vi "labHolo.vi"() -> ()   [LabVIEW 2023] (continued)
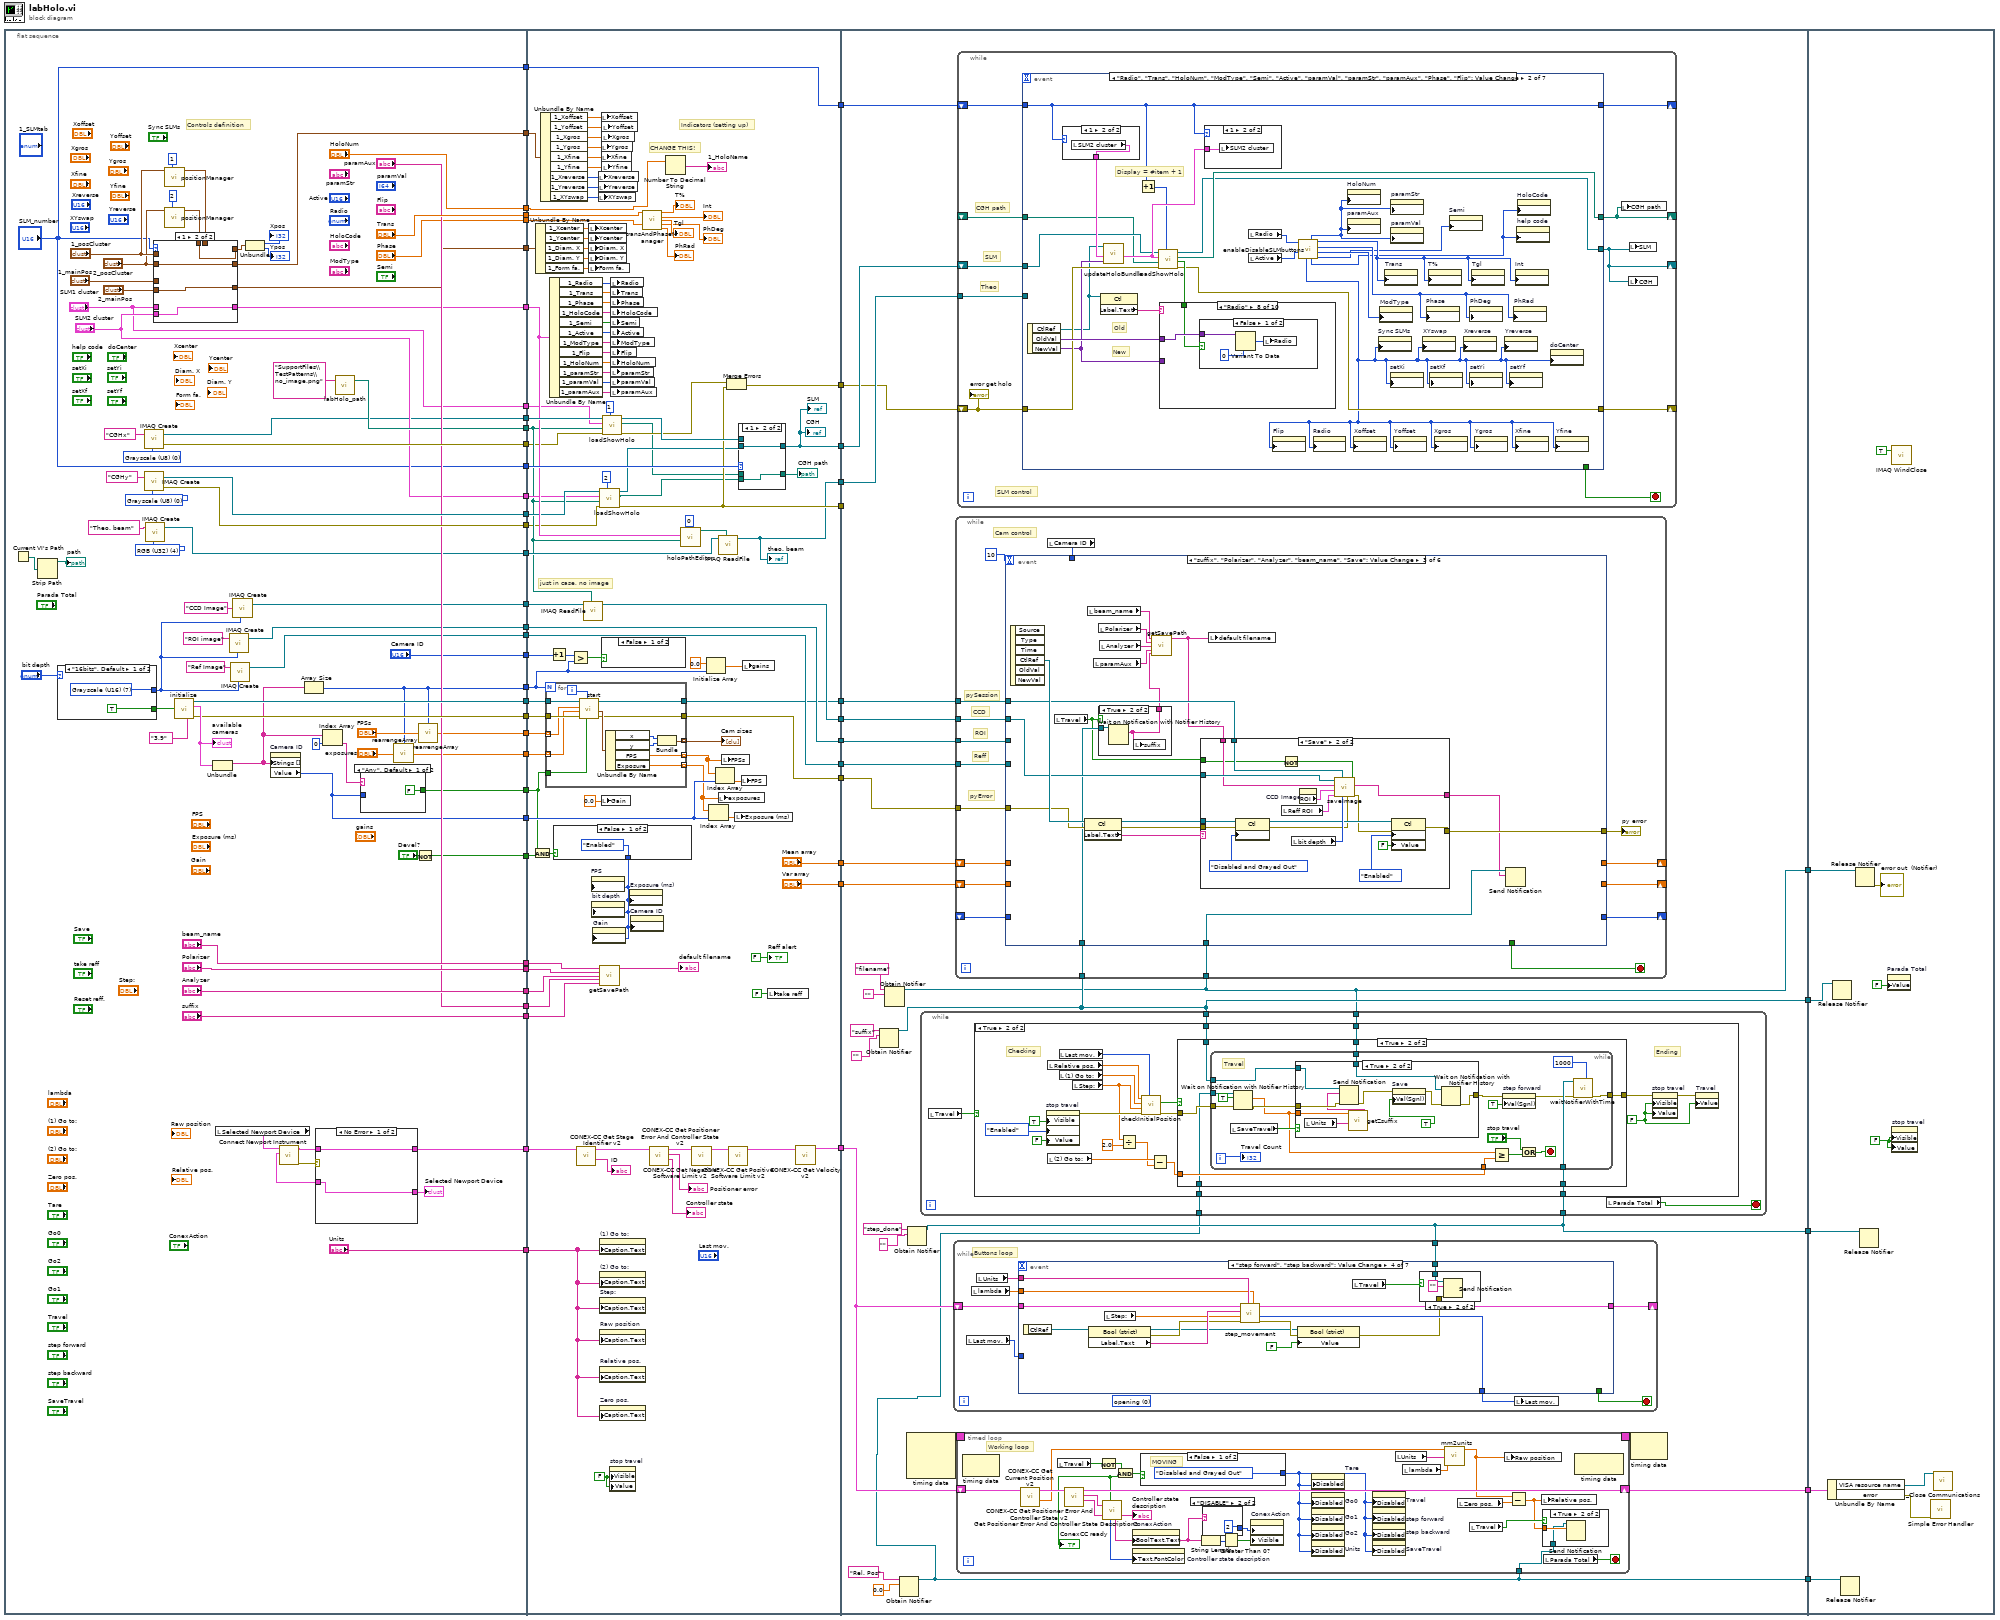
[diagram p0: block diagram]
diagram:
  n1 = flat-sequence {
    tunnel: [w77] -> w53
    tunnel: [w124] -> w52
    tunnel: [w123] -> w51
    tunnel: [w122] -> w50
    tunnel: ["Trans"] -> w47
    tunnel: ["Phase"] -> w46
    tunnel: [w114] -> w45
    tunnel: [w71] -> w44
    tunnel: [w113] -> w43
    tunnel: ["beam_name"] -> w42
    tunnel: ["Polarizer"] -> w41
    tunnel: ["Analyzer"] -> w40
    tunnel: ["suffix"] -> w39
    tunnel: ["paramAux"] -> w38
    tunnel: [w105] -> w37
    tunnel: [w104] -> w35
    tunnel: [w101] -> w33
    tunnel: [w97] -> w32
    tunnel: [w96] -> w31
    tunnel: [w83] -> w30
    tunnel: ["HoloNum"] -> w29
    tunnel: ["SLM1 cluster"] -> w28
    tunnel: [w81] -> w27
    tunnel: ["SLM2 cluster"] -> w26
    tunnel: ["SLM_number"] -> w25
    tunnel: [w74] -> w24
    tunnel: [w65] -> w18
    tunnel: [w63] -> w16
    tunnel: [w70] -> w15
    tunnel: [w68] -> w14
    tunnel: [w66] -> w13
    tunnel: ["Camera ID"] -> w12
    tunnel: ["SLM_number"] -> w10
    tunnel: ["Units"] -> w8
    tunnel: [w57] -> w5
    tunnel: w53 -> [w255]
    tunnel: w52 -> [w200]
    tunnel: w51 -> [w197]
    tunnel: w50 -> [w196]
    tunnel: [w244] -> w49
    tunnel: [w183] -> w48
    tunnel: w47 -> [w249]
    tunnel: w46 -> [w248]
    tunnel: w45 -> [w184]
    tunnel: w44 -> [w181]
    tunnel: w43 -> [w185]
    tunnel: w42 -> [w189]
    tunnel: w41 -> [w188]
    tunnel: w40 -> [w187]
    tunnel: w39 -> [w246]
    tunnel: w38 -> [w186]
    tunnel: w37 -> [w245]
    tunnel: [w243] -> w36
    tunnel: w35 -> [w243]
    tunnel: [w240] -> w34
    tunnel: w33 -> [w240]
    tunnel: w32 -> [w224]
    tunnel: w31 -> [w230]
    tunnel: w30 -> [w207]
    tunnel: w29 -> [w210]
    tunnel: w28 -> [w203]
    tunnel: w27 -> [w198]
    tunnel: w26 -> [w199]
    tunnel: w25 -> [w209]
    tunnel: w24 -> [w208]
    tunnel: [w192] -> w23
    tunnel: [w195] -> w22
    tunnel: [w162] -> w21
    tunnel: ["Mean array"] -> w20
    tunnel: ["Var array"] -> w19
    tunnel: w18 -> [w166]
    tunnel: [w176] -> w17
    tunnel: w16 -> [w175]
    tunnel: w15 -> [w170]
    tunnel: w14 -> [w169]
    tunnel: w13 -> [w174]
    tunnel: w12 -> [w164]
    tunnel: [w158] -> w11
    tunnel: w10 -> [w157]
    tunnel: [w157] -> w9
    tunnel: w8 -> [w155]
    tunnel: [w154] -> w7
    tunnel: w5 -> [w153]
    tunnel: w49 -> [w303]
    tunnel: w48 -> [w302]
    tunnel: w36 -> [w301]
    tunnel: w34 -> [w300]
    tunnel: w23 -> [w296]
    tunnel: w22 -> [_]
    tunnel: w21 -> [w295]
    tunnel: w20 -> [w299]
    tunnel: w19 -> [w298]
    tunnel: w17 -> [w297]
    tunnel: w11 -> [w294]
    tunnel: w9 -> [w293]
    tunnel: w7 -> [w289]
    tunnel: [w290] -> w6
    tunnel: [w282] -> w4
    tunnel: [w281] -> w3
    tunnel: [w280] -> w2
    tunnel: [w277] -> w1
    tunnel: w6 -> [w958]
    tunnel: w4 -> [w955]
    tunnel: w3 -> [w954]
    tunnel: w2 -> [w953]
    tunnel: w1 -> [w952]
    frame #0 {
      w75 = T15 4 items=["Grayscale (U8)", "Grayscale (I16)", "Grayscale (SGL)", "Complex (CSG)", "RGB (U32)", "HSL (U32)", "RGB (U64)", "Grayscale (U16)"] ("Image Type")
      w117 = T15 0 items=["Grayscale (U8)", "Grayscale (I16)", "Grayscale (SGL)", "Complex (CSG)", "RGB (U32)", "HSL (U32)", "RGB (U64)", "Grayscale (U16)"] ("Image Type")
      w118 = T15 0 items=["Grayscale (U8)", "Grayscale (I16)", "Grayscale (SGL)", "Complex (CSG)", "RGB (U32)", "HSL (U32)", "RGB (U64)", "Grayscale (U16)"] ("Image Type")
      # "Controls definition"
      n2 = Current VI's Path() -> (path=w121:path)
      n3 = Strip Path(path=w121) -> (stripped path=→"path":path)  [unwired: 1 out]
      n4 = case shown="\"16bits\", Default" "bit depth" {
        tunnel: [w143 w145] -> w102
        tunnel: [TRUE FALSE] -> w107
        frame "16bits", Default {
          w143 = T15 7 items=["Grayscale (U8)", "Grayscale (I16)", "Grayscale (SGL)", "Complex (CSG)", "RGB (U32)", "HSL (U32)", "RGB (U64)", "Grayscale (U16)"] ("Image Type")
        }
        frame "8bits" {
          w145 = T15 0 items=["Grayscale (U8)", "Grayscale (I16)", "Grayscale (SGL)", "Complex (CSG)", "RGB (U32)", "HSL (U32)", "RGB (U64)", "Grayscale (U16)"] ("Image Type")
        }
      }
      n5 = call "IMAQ Create"("Image Name"="CGHx", "Image Type"=w118) -> ("New Image"=w77:T6, "error out"=w122:errorcluster)  [unwired: 3 in]
      n6 = call "IMAQ Create"("Image Name"="CGHy", "Image Type"=w117) -> ("New Image"=w124:T6, "error out"=w123:errorcluster)  [unwired: 3 in]
      n7 = call "IMAQ Create"("Image Name"="Theo. beam", "Image Type"=w75) -> ("New Image"=w74:T6)  [unwired: 3 in, 1 out]
      n8 = call "positionManager.vi"("Display"=1, "Cluster"="1_posCluster") -> ("output cluster"=w89:cluster{i32, i32})  [unwired: 5 in, 2 out]
      n9 = call "positionManager.vi"("Display"=2, "Cluster"="2_posCluster") -> ("output cluster"=w90:cluster{i32, i32})  [unwired: 5 in, 2 out]
      n10 = case shown="1" "SLM_number" {
        tunnel: [w135 w137] -> w97
        tunnel: [w134 w139] -> w96
        tunnel: "1_posCluster" -> [w135 _]
        tunnel: "1_mainPos" -> [w134 _]
        tunnel: "2_posCluster" -> [_ w137]
        tunnel: "2_mainPos" -> [_ w139]
        tunnel: "SLM1 cluster" -> [w133 _]
        tunnel: "SLM2 cluster" -> [_ w138]
        tunnel: [w133 w138] -> w83
        tunnel: [w132 w136] -> w84
        tunnel: w90 -> [_ w136]
        tunnel: w89 -> [w132 _]
        frame 0, Default {
        }
        frame 1 {
        }
      }
      n11 = call "initialize.vi"("14bits"=w107, "sys Python version"="3.9") -> ("session out"=w113:refnum<k35>, "available cameras"=w115:cluster{string[], string[]}, "error out"=w114:errorcluster)  [unwired: 2 in]
      "available\ncameras" <- w115
      n12 = Unbundle(w115) -> (w99:string[])  [unwired: 1 out]
      n13 = local read "Selected Newport Device"() -> (w59:T1)
      n14 = call "IMAQ Create"("Image Name"="ROI image", "Image Type"=w102) -> ("New Image"=w101:T6)  [unwired: 3 in, 1 out]
      n15 = call "IMAQ Create"("Image Name"="Ref Image", "Image Type"=w102) -> ("New Image"=w104:T6)  [unwired: 3 in, 1 out]
      n16 = call "IMAQ Create"("Image Name"="CCD Image", "Image Type"=w102) -> ("New Image"=w105:T6)  [unwired: 3 in, 1 out]
      n17 = Unbundle(w84) -> (→"Xpos":i32, →"Ypos":i32)
      n18 = property on="Camera ID" class="Ring (strict)"("Strings []"=w99) -> ("Value"=w71:u16)  [unwired: 2 in, 2 out]
      n19 = call "Connect Newport Instrument.vi"("Selected Device Cluster (INPUT)"=w59) -> ("error (duplicate)"=w58:errorcluster, "Device Connection Cluster"=w56:T16, "Selected Device Cluster (OUTPUT)"=w55:T1)  [unwired: 5 in, 3 out]
      n20 = Array Size(array=w99) -> (size(s)=w65:i32)
      n21 = case shown="No Error" w58 {
        tunnel: [w128 w131] -> w57
        tunnel: w56 -> [w128 _]
        tunnel: w55 -> [w127 _]
        tunnel: [w127 w129] -> w54
        frame No Error {
        }
        frame Error {
          n22 = call "Connect Newport Instrument.vi"("Selected Device Cluster (INPUT)"=T10 {"Found resources names"=["ASRL1::INSTR", "ASRL3::INSTR"], "Found interfaces names"=["ASRL1  (COM1 - Puerto de comunicaciones)", "ASRL3  (COM3 - USB Serial Port)"], "OK?"=FALSE, "Selected device"="", "Address"=0, "error"={"status"=TRUE, "code"=0, "source"=""}}) -> ("Device Connection Cluster"=w131:T16, "Selected Device Cluster (OUTPUT)"=w129:T1)  [unwired: 5 in, 4 out]
        }
      }
      "Selected Newport Device" <- w54
      n23 = Index Array(array=w99, index=0) -> (element=w100:string)
      n24 = call "labHolo_path.vi"("sub folder or file (str)"="SupportFiles\\TestPatterns\\no_image.png") -> ("labHolo path"=w81:path)  [unwired: 1 in, 1 out]
      n25 = case shown="\"Any\", Default" w100 {
        tunnel: w71 -> [_ _]
        tunnel: [FALSE TRUE] -> w70
        frame "Any", Default {
        }
        frame "NotFound" {
        }
      }
      n26 = call "rearrengeArray.vi"("array in"="exposures", "desired size"=w65) -> ("array out"=w63:dbl[])
      n27 = Not(x="Devel?") -> (.not. x?=w68:bool)
      n28 = call "rearrengeArray.vi"("array in"="FPSs", "desired size"=w65) -> ("array out"=w66:dbl[])
    }
    frame #1 {
      w146 = FALSE ("Visible")
      # "just in case, no image"
      # "CHANGE THIS!"
      # "Indicators (setting up)"
      n29 = And(x=w170, y=w169) -> (x .and. y?=w171:bool)
      n30 = Unbundle By Name(w230) -> ("1_Xcenter"=w229:dbl, "1_Ycenter"=w228:dbl, "1_Diam. X"=w227:dbl, "1_Diam. Y"=w226:dbl, "1_Form fa."=w225:dbl)
      n31 = Unbundle By Name(w224) -> ("1_Xoffset"=w239:dbl, "1_Yoffset"=w238:dbl, "1_Xgros"=w237:dbl, "1_Ygros"=w236:dbl, "1_Xfine"=w235:dbl, "1_Yfine"=w234:dbl, "1_Xreverse"=w233:u16, "1_Yreverse"=w232:u16, "1_XYswap"=w231:u16)
      n32 = for {
        N: w166 -> [_]
        tunnel: w185 -> [w272]
        tunnel: w184 -> [w271]
        tunnel: [w270] -> w183
        tunnel: [w269] -> w179 mode=indexing
        tunnel: [w268] -> w180 mode=indexing
        tunnel: [w266] -> w177 mode=indexing
        tunnel: [w265] -> w176
        tunnel: w174 -> [w264] mode=indexing
        tunnel: w175 -> [w263] mode=indexing
        tunnel: w170 -> [w259]
        i -> [w262]
        n33 = call "start.vi"("Not found"=w259, "Cam id"=w262, "error in (no error)"=w271, "Exposure (ms)"=w263, "FPS"=w264, "session in"=w272) -> ("error out"=w265:errorcluster, "cam attr."=w267:T17, "session out"=w270:refnum<k35>)  [unwired: 2 in]
        n34 = Unbundle By Name(w267) -> ("x"=w261:i32, "y"=w260:i32, "FPS"=w269:dbl, "Exposure"=w268:dbl)
        n35 = Bundle("x"=w261, "y"=w260) -> (w266:cluster{"x":i32, "y":i32})  [unwired: 1 in]
      }
      "Cam sizes" <- w177
      n36 = Unbundle By Name(w207) -> ("1_Radio"=w223:T7, "1_Trans"=w222:dbl, "1_Phase"=w221:dbl, "1_HoloCode"=w220:string, "1_Semi"=w219:bool, "1_Active"=w218:u16, "1_ModType"=w217:string, "1_Flip"=w216:string, "1_HoloNum"=w215:dbl, "1_paramStr"=w214:string, "1_paramVal"=w213:i64, "1_paramAux"=w212:string)
      n37 = Increment(x=w164) -> (x+1=w165:u16)
      n38 = case shown="False" w171 {
        tunnel: [T11."Enabled" ("Disabled") T11."Disabled and Grayed Out" ("Disabled")] -> w163
        frame False {
        }
        frame True {
        }
      }
      n39 = Greater?(x=w165, y=w166) -> (0:w167:bool)
      n40 = call "CONEX-CC Get Stage Identifier v2.vi"("Connection Cluster in"=w153) -> ("Identifier"=→"ID":string, "Connection Cluster out"=w149:T16)  [unwired: 9 in]
      n41 = call "IMAQ ReadFile"("File Path"=w198, "Image"=w245) -> ("Image Out"=w244:T6)  [unwired: 5 in, 4 out]
      n42 = local write "Xcenter"(w229) -> ()
      n43 = local write "Ycenter"(w228) -> ()
      n44 = local write "Diam. X"(w227) -> ()
      n45 = local write "Diam. Y"(w226) -> ()
      n46 = local write "Form fa."(w225) -> ()
      n47 = property on="FPS" class="DigNum (strict)"("DisabledEnum"=w163) -> ()  [unwired: 2 in, 2 out]
      n48 = property on="bit depth" class="Enum (strict)"("DisabledEnum"=w163) -> ()  [unwired: 2 in, 2 out]
      n49 = property on="Gain" class="DigNum (strict)"("DisabledEnum"=w163) -> ()  [unwired: 2 in, 2 out]
      n50 = local write "Xreverse"(w233) -> ()
      n51 = local write "Yreverse"(w232) -> ()
      n52 = local write "XYswap"(w231) -> ()
      n53 = call "loadShowHolo.vi"("Display"=u16 2, "error in (no error)"=w197, "prev. path"=w198, "SLM1 cluster"=w199, "Image in"=w200) -> ("error out"=w195:errorcluster, "appended path"=w159:path, "Image out"=w193:T6)  [unwired: 3 in, 1 out]
      n54 = call "getSavePath.vi"("beam_name"=w189, "Polarizer"=w188, "Analyzer"=w187, "prefix"=w186, "suffix"=w246) -> ("appended filename"=→"default filename":string)  [unwired: 10 in]
      n55 = property on="(1) Go to:" class="DigNum (strict)"("Caption.Text"=w155) -> ()  [unwired: 2 in, 2 out]
      n56 = property on="(2) Go to:" class="DigNum (strict)"("Caption.Text"=w155) -> ()  [unwired: 2 in, 2 out]
      n57 = property on="Step:" class="DigNum (strict)"("Caption.Text"=w155) -> ()  [unwired: 2 in, 2 out]
      n58 = property on="Raw position" class="DigNum (strict)"("Caption.Text"=w155) -> ()  [unwired: 2 in, 2 out]
      n59 = property on="Relative pos." class="DigNum (strict)"("Caption.Text"=w155) -> ()  [unwired: 2 in, 2 out]
      n60 = property on="Zero pos." class="DigNum (strict)"("Caption.Text"=w155) -> ()  [unwired: 2 in, 2 out]
      n61 = local write "Xoffset"(w239) -> ()
      n62 = local write "Ygros"(w236) -> ()
      n63 = local write "Xfine"(w235) -> ()
      n64 = local write "Gain"(0.0 ("Gain")) -> ()
      n65 = local write "Yoffset"(w238) -> ()
      n66 = local write "Xgros"(w237) -> ()
      n67 = local write "Yfine"(w234) -> ()
      n68 = case shown="False" w167 {
        frame False {
        }
        frame True {
          n69 = local write "Camera ID"(u16 0) -> ()
        }
      }
      n70 = call "loadShowHolo.vi"("Display"=u16 1, "error in (no error)"=w196, "prev. path"=w198, "SLM1 cluster"=w203, "Image in"=w255) -> ("error out"=w161:errorcluster, "appended path"=w160:path, "Image out"=w202:T6)  [unwired: 3 in, 1 out]
      n71 = property on="stop travel" class="Bool (strict)"("Visible"=w146, "Value"=w146) -> ()  [unwired: 2 in, 2 out]
      n72 = local write "Radio"(w223) -> ()
      n73 = local write "Trans"(w222) -> ()
      n74 = local write "Phase"(w221) -> ()
      n75 = local write "HoloCode"(w220) -> ()
      n76 = local write "Semi"(w219) -> ()
      n77 = local write "Active"(w218) -> ()
      n78 = local write "ModType"(w217) -> ()
      n79 = local write "Flip"(w216) -> ()
      n80 = local write "HoloNum"(w215) -> ()
      n81 = local write "paramStr"(w214) -> ()
      n82 = local write "paramVal"(w213) -> ()
      n83 = local write "paramAux"(w212) -> ()
      n84 = property on="Exposure (ms)" class="DigNum (strict)"("DisabledEnum"=w163) -> ()  [unwired: 2 in, 2 out]
      n85 = property on="Camera ID" class="Ring (strict)"("DisabledEnum"=w163) -> ()  [unwired: 2 in, 2 out]
      n86 = call "transAndPhaseManager.vi"("Trans in"=w249, "Phase in"=w248) -> ("Trans %"=→"T%":dbl, "Intensity"=→"Int":dbl, "T gl"=→"Tgl":dbl, "Phase Deg"=→"PhDeg":dbl, "Phase Rad"=→"PhRad":dbl)  [unwired: 9 in]
      n87 = call "CONEX-CC Get Positioner Error And Controller State v2.vi"("Connection Cluster in"=w149) -> ("Controller state"=→"Controller state":string, "Positioner error"=→"Positioner error":string, "Connection Cluster out"=w148:T16)  [unwired: 8 in]
      n88 = Number To Decimal String(number=w210) -> (decimal integer string=→"1_HoloName":string)  [unwired: 1 in]
      n89 = call "holoPathEditor.vi"("Display"=u16 0, "prev. Path"=w198, "input cluster"=w207) -> ("appended path"=w206:path)  [unwired: 5 in, 3 out]
      n90 = call "CONEX-CC Get Negative Software Limit v2.vi"("Connection Cluster in"=w148) -> ("Connection Cluster out"=w147:T16)  [unwired: 9 in, 1 out]
      n91 = Initialize Array(0.0 ("element"), w166) -> (w173:dbl[])
      n92 = Index Array(array=w180, index=w181) -> (element=w178:dbl)
      n93 = Index Array(array=w179, index=w181) -> (element=w182:dbl)
      n94 = call "IMAQ ReadFile"("File Path"=w206, "Image"=w208) -> ("Image Out"=w162:T6)  [unwired: 5 in, 4 out]
      "theo. beam" <- w162
      n95 = local write "exposures"(w180) -> ()
      n96 = local write "FPSs"(w179) -> ()
      n97 = Merge Errors(w161, w195) -> (w158:errorcluster)
      n98 = call "CONEX-CC Get Positive Software Limit v2.vi"("Connection Cluster in"=w147) -> ("Connection Cluster out"=w156:T16)  [unwired: 9 in, 1 out]
      n99 = local write "Exposure (ms)"(w178) -> ()
      n100 = case shown="1" w209 {
        tunnel: [w274 w276] -> w192
        tunnel: w202 -> [w274 _]
        tunnel: w160 -> [w273 _]
        tunnel: [w273 w275] -> w194
        tunnel: w193 -> [_ w276]
        tunnel: w159 -> [_ w275]
        frame 0, Default {
        }
        frame 1 {
        }
      }
      "CGH path" <- w194
      "CGH" <- w192
      "SLM" <- w192
      n101 = local write "FPS"(w182) -> ()
      n102 = local write "gains"(w173) -> ()
      n103 = local write "take reff"(FALSE ("take reff")) -> ()
      n104 = call "CONEX-CC Get Velocity v2.vi"("Connection Cluster in"=w156) -> ("Connection Cluster out"=w154:T16)  [unwired: 8 in, 2 out]
      "Reff alert" <- FALSE ("Boolean")
    }
    frame #2 {
      n105 = Obtain Notifier(name (unnamed)="suffix", notification data type="") -> (notifier out=w281:refnum<notifier>)  [unwired: 2 in, 2 out]
      n106 = Obtain Notifier(name (unnamed)="filename", notification data type="") -> (notifier out=w280:refnum<notifier>)  [unwired: 2 in, 2 out]
      n107 = Obtain Notifier(name (unnamed)="Rel. Pos", notification data type=0.0) -> (notifier out=w277:refnum<notifier>)  [unwired: 2 in, 2 out]
      n108 = node-c288() -> (w292:T12)  [unwired: 2 in, 1 out]
      n109 = Obtain Notifier(name (unnamed)="step_done", notification data type="") -> (notifier out=w282:refnum<notifier>)  [unwired: 2 in, 2 out]
      n110 = while {
        tunnel: w281 -> [w307]
        tunnel: w282 -> [w306]
        tunnel: w280 -> [w305]
        tunnel: w277 -> [w304]
        stop <- w308 stop-if-true
        n111 = local read "Travel"() -> (w309:bool)
        n112 = case shown="True" w309 {
          tunnel: w307 -> [_ w330]
          tunnel: w306 -> [_ w329]
          tunnel: w305 -> [_ w311]
          tunnel: w304 -> [_ w310]
          frame False {
          }
          frame True {
            w318 = FALSE ("Visible")
            # "Ending"
            # "Checking"
            n113 = property on="stop travel" class="Bool (strict)"("Visible"=TRUE, "DisabledEnum"=T11."Enabled" ("Disabled"), "Value"=FALSE ("stop travel")) -> (error out=w325:errorcluster)  [unwired: 2 in, 1 out]
            n114 = local read "Relative pos."() -> (w322:dbl)
            n115 = local read "(2) Go to:"() -> (w316:dbl)
            n116 = local read "Last mov."() -> (w323:u16)
            n117 = local read "(1) Go to:"() -> (w324:dbl)
            n118 = local read "Step:"() -> (w314:dbl)
            n119 = Divide(x=w314, y=2.0) -> (x/y=w312:dbl)
            n120 = call "checkInitialPosition.vi"("Last mov."=w323, "error in (no error)"=w325, "Step"=w314, "Initial pos"=w324, "Current pos"=w322) -> ("error out"=w321:errorcluster, "go"=w317:bool)  [unwired: 5 in]
            n121 = Subtract(x=w316, y=w312) -> (x-y=w315:dbl)
            n122 = case shown="True" w317 {
              tunnel: w330 -> [_ w338]
              tunnel: w329 -> [_ w337]
              tunnel: w321 -> [w331 w336]
              tunnel: [w331 w335] -> w320
              tunnel: w315 -> [_ w334]
              tunnel: w311 -> [_ w333]
              tunnel: w310 -> [_ w332]
              frame False {
              }
              frame True {
                n123 = while {
                  tunnel: w338 -> [w354]
                  tunnel: w337 -> [w343]
                  tunnel: w336 -> [w347]
                  tunnel: [w341] -> w335
                  tunnel: w334 -> [w352]
                  tunnel: w333 -> [w348]
                  tunnel: w332 -> [w345]
                  i -> [w353]
                  stop <- w357 stop-if-true
                  # "Travel"
                  n124 = local read "SaveTravel"() -> (w356:bool)
                  n125 = Wait on Notification with Notifier History(0:w345, 1:TRUE ("ignore previous (F)"), 3:w347) -> (9:w344:dbl, 11:w346:errorcluster)  [unwired: 1 in, 2 out]
                  n126 = case shown="True" w356 {
                    tunnel: w346 -> [w358 w364]
                    tunnel: [w358 w359] -> w349
                    tunnel: w354 -> [_ w362]
                    tunnel: w344 -> [_ w366]
                    tunnel: w348 -> [_ w361]
                    frame False {
                    }
                    frame True {
                      n127 = local read "Units"() -> (w367:string)
                      n128 = call "getZsuffix.vi"("Units"=w367, "Zposition"=w366) -> ("String"=w363:string)  [unwired: 9 in]
                      n129 = Send Notification(notification=w363, notifier=w362, error in (no error)=w364) -> (error out=w365:errorcluster)  [unwired: 1 out]
                      n130 = property on="Save" class="Bool (strict)"(error in=w365, "Val(Sgnl)"=TRUE ("Value (Signaling)")) -> (error out=w360:errorcluster)  [unwired: 1 in, 1 out]
                      n131 = Wait on Notification with Notifier History(0:w361, 3:w360) -> (11:w359:errorcluster)  [unwired: 2 in, 3 out]
                    }
                  }
                  n132 = Greater Or Equal?(x=w344, y=w352) -> (x >= y?=w350:bool)
                  n133 = property on="step forward" class="Bool (strict)"(error in=w349, "Val(Sgnl)"=TRUE ("Value (Signaling)")) -> (error out=w342:errorcluster)  [unwired: 1 in, 1 out]
                  n134 = Or(x="stop travel", y=w350) -> (x .or. y?=w357:bool)
                  n135 = call "waitNotifierWithTime.vi"("min wait in ms (500)"=u32 1000 ("min wait in ms (300)"), "error in (no error)"=w342, "Notifier in"=w343) -> ("error out"=w341:errorcluster)  [unwired: 6 in, 2 out]
                  "Travel Count" <- w353
                }
              }
            }
            n136 = property on="stop travel" class="Bool (strict)"(error in=w320, "Visible"=w318, "Value"=w318) -> (error out=w319:errorcluster)  [unwired: 1 in, 1 out]
            n137 = property on="Travel" class="Bool (strict)"(error in=w319, "Value"=w318) -> ()  [unwired: 1 in, 2 out]
          }
        }
        n138 = local read "Parada Total"() -> (w308:bool)
      }
      n139 = while {
        shift-right: [w409] -> _
        shift-left: w289 -> [w410]
        tunnel: w282 -> [w404]
        stop <- w411 stop-if-true
        (unwired) u16 0 items=["opening", "homing", "toLeft", "toRight", "closing"] ("Last movement")
        # "Buttons loop"
        n140 = local read "Last mov."() -> (w405:u16)
        n141 = local read "lambda"() -> (w407:dbl)
        n142 = local read "Units"() -> (w408:string)
        n143 = event shown="[3] \"step forward\", \"step backward\": Value Change" {
          selector: _ -> [_ _ _ _ _ _ _]
          dyn-events: _ -> [_ _ _ _ _ _ _]
          timeout: _ -> [_ _ _ _ _ _ _]
          tunnel: [_ w415 _ _ _ _ _] -> w411
          tunnel: w410 -> [_ w416 w434 w468 w488 w495 w506]
          tunnel: [_ w414 w433 w467 w487 w495 w506] -> w409
          tunnel: w408 -> [_ _ _ w461 w486 _ _]
          tunnel: w407 -> [_ _ _ w460 w485 _ w499]
          tunnel: [w412 w413 w429 w458 w477 w494 w498] -> w406
          tunnel: w405 -> [w412 w413 w428 _ _ w494 w498]
          tunnel: w404 -> [_ _ _ w459 _ _ _]
          event Timeout {
            n144 = event-data() -> ()  [unwired: 1 in, 3 out]
          }
          event "Parada Total": Value Change {
            n145 = event-data() -> ()  [unwired: 1 in, 1 out]
            n146 = flat-sequence {
              tunnel: [w421] -> w419
              tunnel: w416 -> [w420]
              tunnel: w419 -> [w423]
              tunnel: [w423] -> w418
              tunnel: w418 -> [w425]
              tunnel: [w425] -> w417
              tunnel: [w427] -> w414
              tunnel: w417 -> [w427]
              tunnel: [TRUE] -> w415
              frame #0 {
                n147 = call "CONEX-CC Stop Motion v2.vi"("Connection Cluster in"=w420) -> ("Connection Cluster out"=w421:T16)  [unwired: 10 in]
              }
              frame #1 {
                n148 = local write "Travel"(FALSE) -> ()
              }
              frame #2 {
                n149 = Wait (ms)(milliseconds to wait=u32 200 ("attente (ms)")) -> ()  [unwired: 1 out]
              }
              frame #3 {
              }
            }
          }
          event "ConexAction": Value Change {
            n150 = event-data() -> ("CtlRef"=w431:refnum<vi>)  [unwired: 1 in]
            n151 = property on="Property Node" class="Bool (strict)"(reference=w431) -> ("BoolText.Text"=w430:string)  [unwired: 1 in, 2 out]
            n152 = case shown="\"STOP\"" w430 {
              tunnel: w434 -> [w437 w440 w443 w451 w454]
              tunnel: [w436 w440 w442 w450 w455] -> w433
              tunnel: [w435 w439 w441 w448 w453] -> w429
              tunnel: w428 -> [w435 w439 _ w448 w453]
              frame "ENABLE" {
                n153 = call "CONEX-CC Enter-Leave DISABLE State v2.vi"("Ready? (false=DISABLE true=READY)"=TRUE ("Flag (false=DISABLE true=READY)"), "Connection Cluster in"=w437) -> ("Connection Cluster out"=w436:T16)  [unwired: 7 in]
              }
              frame Default {
              }
              frame "HOME" {
                n154 = flat-sequence {
                  tunnel: w443 -> [w447]
                  tunnel: [w446] -> w442
                  tunnel: [w445] -> w441
                  frame #0 {
                    n155 = One Button Dialog(message="The Stage will go to the 0 position. Check that the travel is clean!") -> ()  [unwired: 1 in, 1 out]
                  }
                  frame #1 {
                    w445 = u16 0 items=["opening", "homing", "toLeft", "toRight", "closing"] ("Last movement")
                    n156 = call "CONEX-CC Home search v2.vi"("Connection Cluster in"=w447) -> ("Connection Cluster out"=w446:T16)  [unwired: 5 in, 3 out]
                  }
                }
              }
              frame "DISABLE" {
                n157 = call "CONEX-CC Enter-Leave DISABLE State v2.vi"("Ready? (false=DISABLE true=READY)"=FALSE ("Flag (false=DISABLE true=READY)"), "Connection Cluster in"=w451) -> ("Connection Cluster out"=w450:T16)  [unwired: 7 in]
              }
              frame "STOP" {
                n158 = call "CONEX-CC Stop Motion v2.vi"("Connection Cluster in"=w454) -> ("Connection Cluster out"=w455:T16)  [unwired: 10 in]
                n159 = local write "stop travel"(TRUE ("stop travel")) -> ()
              }
            }
            n160 = property on="ConexAction" class="Bool (strict)"("Value"=FALSE) -> ()  [unwired: 2 in, 2 out]
          }
          event "step forward", "step backward": Value Change {
            n161 = event-data() -> ("CtlRef"=w470:refnum<vi>)  [unwired: 1 in]
            n162 = property on="Property Node" class="Bool (strict)"(reference=w470) -> (reference out=w463:refnum<vi>, error out=w465:errorcluster, "Label.Text"=w466:string)  [unwired: 1 in]
            n163 = local read "Step:"() -> (w462:dbl)
            n164 = call "step_movement.vi"("lambda (nm)"=w460, "Units"=w461, "error in (no error)"=w465, "step (units)"=w462, "Step type (fordward)"=w466, "Connection Cluster in"=w468) -> ("error out"=w464:errorcluster, "Last mov."=w458:u16, "Connection Cluster out"=w467:T16)  [unwired: 3 in]
            n165 = property on="Property Node" class="Bool (strict)"(reference=w463, error in=w464, "Value"=FALSE) -> (error out=w457:errorcluster)  [unwired: 1 out]
            n166 = local read "Travel"() -> (w456:bool)
            n167 = case shown="True" w456 {
              tunnel: w459 -> [_ w473]
              tunnel: w457 -> [_ w472]
              frame False {
              }
              frame True {
                n168 = Send Notification(notification="", notifier=w473, error in (no error)=w472) -> ()  [unwired: 2 out]
              }
            }
          }
          event "Go1", "Go2", "Go0": Value Change {
            n169 = event-data() -> ("CtlRef"=w484:refnum<vi>)  [unwired: 1 in]
            n170 = property on="Property Node" class="Bool (strict)"(reference=w484) -> (reference out=w483:refnum<vi>, "Label.Text"=w481:string)  [unwired: 1 in, 1 out]
            n171 = case shown="\"Go0\", Default" w481 {
              tunnel: [w491 w492 0.0 ("(2) Go to:")] -> w475
              frame "Go1" {
                n172 = local read "(1) Go to:"() -> (w491:dbl)
              }
              frame "Go2" {
                n173 = local read "(2) Go to:"() -> (w492:dbl)
              }
              frame "Go0", Default {
              }
            }
            n174 = local read "Zero pos."() -> (w476:dbl)
            n175 = Add(x=w476, y=w475) -> (x+y=w474:dbl)
            n176 = local read "Relative pos."() -> (w479:dbl)
            n177 = call "units2mm.vi"("lambda (nm)"=w485, "target units"=w486, "position in units"=w474) -> ("raw postion (mm)"=w480:dbl)  [unwired: 8 in]
            n178 = property on="Property Node" class="Bool (strict)"(reference=w483, "Value"=FALSE) -> ()  [unwired: 1 in, 2 out]
            n179 = Greater?(x=w480, y=w479) -> (0:w478:bool)
            n180 = case shown="False" w478 {
              tunnel: [w489 w490] -> w477
              frame False {
                w489 = u16 2 items=["opening", "homing", "toLeft", "toRight", "closing"] ("Last movement")
              }
              frame True {
                w490 = u16 3 items=["opening", "homing", "toLeft", "toRight", "closing"] ("Last movement")
              }
            }
            n181 = call "CONEX-CC Absolute Move v2.vi"("Target position"=w480, "Connection Cluster in"=w488) -> ("Connection Cluster out"=w487:T16)  [unwired: 5 in, 2 out]
          }
          event "Tare": Value Change {
            n182 = event-data() -> ()  [unwired: 1 in, 2 out]
            n183 = local read "Raw position"() -> (w497:dbl)
            n184 = local write "Tare"(FALSE ("Tare")) -> ()
            n185 = local write "Zero pos."(w497) -> ()
          }
          event "Units": Value Change {
            n186 = event-data() -> ("OldVal"=w505:string, "NewVal"=w507:string)  [unwired: 1 in]
            n187 = property on="(1) Go to:" class="DigNum (strict)"("Caption.Text"=w507) -> ()  [unwired: 2 in, 2 out]
            n188 = property on="(2) Go to:" class="DigNum (strict)"("Caption.Text"=w507) -> ()  [unwired: 2 in, 2 out]
            n189 = property on="Zero pos." class="DigNum (strict)"("Caption.Text"=w507) -> ()  [unwired: 2 in, 2 out]
            n190 = property on="Raw position" class="DigNum (strict)"("Caption.Text"=w507) -> ()  [unwired: 2 in, 2 out]
            n191 = property on="Relative pos." class="DigNum (strict)"("Caption.Text"=w507) -> ()  [unwired: 2 in, 2 out]
            n192 = property on="Step:" class="DigNum (strict)"("Caption.Text"=w507) -> ()  [unwired: 2 in, 2 out]
            n193 = case shown="\"lam\"" w507 {
              tunnel: [1000000.0 1000.0 1.0 w515] -> w500
              tunnel: w499 -> [_ _ _ w515]
              frame "mm", Default {
              }
              frame "um" {
              }
              frame "nm" {
              }
              frame "lam" {
              }
            }
            n194 = case shown="\"lam\"" w505 {
              tunnel: [1000000.0 1000.0 1.0 w511] -> w501
              tunnel: w499 -> [_ _ _ w511]
              frame "mm", Default {
              }
              frame "um" {
              }
              frame "nm" {
              }
              frame "lam" {
              }
            }
            n195 = Divide(x=w501, y=w500) -> (x/y=w502:dbl)
            n196 = local read "Zero pos."() -> (w504:dbl)
            n197 = Multiply(x=w504, y=w502) -> (x*y=w503:dbl)
            n198 = local write "Zero pos."(w503) -> ()
          }
        }
        n199 = local write "Last mov."(w406) -> ()
      }
      n200 = while {
        shift-right: [w809] -> _
        shift-left: _ -> [w808]
        tunnel: w303 -> [w806]
        tunnel: w302 -> [w805]
        tunnel: w301 -> [w803]
        tunnel: w300 -> [w802]
        shift-right: [w798] -> _
        shift-left: w299 -> [w800]
        shift-right: [w797] -> _
        shift-left: w298 -> [w799]
        tunnel: w297 -> [w796]
        tunnel: w280 -> [w795]
        tunnel: w281 -> [w794]
        stop <- w810 stop-if-true
        # "Cam control"
        # "pyError"
        # "Reff"
        # "ROI"
        # "CCD"
        # "pySession"
        n201 = local read "Camera ID"() -> (w801:u16)
        n202 = event shown="[2] \"suffix\", \"Polarizer\", \"Analyzer\", \"beam_name\", \"Save\": Value Change" {
          selector: _ -> [_ _ _ _ _ _]
          dyn-events: _ -> [_ _ _ _ _ _]
          timeout: 10 -> [_ _ _ _ _ _]
          tunnel: [_ _ _ _ _ w951] -> w810
          tunnel: [w835 _ _ _ _ _] -> w809
          tunnel: w808 -> [w844 _ _ _ _ _]
          tunnel: w806 -> [w842 _ w864 _ _ _]
          tunnel: w805 -> [w841 _ w863 w906 _ _]
          tunnel: [w840 _ w862 w904 _ _] -> w804
          tunnel: w803 -> [w821 _ _ _ _ _]
          tunnel: w802 -> [w820 _ _ _ _ _]
          tunnel: w801 -> [w822 _ _ w895 _ _]
          tunnel: w800 -> [w816 _ _ _ _ _]
          tunnel: w799 -> [w815 _ _ _ _ _]
          tunnel: [w814 _ _ _ _ _] -> w798
          tunnel: [w813 _ _ _ _ _] -> w797
          tunnel: w796 -> [w811 _ w860 w894 _ _]
          tunnel: w795 -> [_ _ w857 _ _ _]
          tunnel: w794 -> [_ _ w855 _ _ _]
          event Timeout {
            n203 = event-data() -> ()  [unwired: 1 in, 3 out]
            n204 = call "capture.vi"("error in (no error)"=w811, "Cam ID"=w822, "Image in"=w842, "session in"=w841) -> ("error out"=w840:errorcluster, "Image out"=w819:T6)  [unwired: 3 in, 1 out]
            n205 = local read "bit depth"() -> (w826:enum16{"16bits", "14bits", "12bits", "8bits"})
            n206 = property on="CCD Image" class="ImageControl"() -> ("ROI"=w827:T8)  [unwired: 2 in, 2 out]
            "ROI" <- w827
            n207 = call "histogram.vi"("Image ROI"=w820, "useROI"="Whole/ROI", "ROI Descriptor"=w827, "bit depth"=w826, "Image"=w819) -> ("Statistics"=w832:T18, "Histograph"=→"Histograph":T9, "bins"=w817:i32)  [unwired: 2 in, 2 out]
            n208 = Unbundle By Name(w832) -> ("mean (ROI)"=→"mean bar" →"mean":dbl, "max (ROI)"=→"max":i16, "max_counts"=w829:dbl, "image_size"=→"ROI size":i32, "# Sat. Pixels"=→"# Sat. Pixels":sgl)
            n209 = control-ref of="Histograph"() -> (w828:refnum<vi>)
            n210 = control-ref of="Reff ROI"() -> (w833:refnum<vi>)
            n211 = call "setHistogram.vi"("Auto. In"="Auto. hist", "max counts"=w829, "bins"=w817, "WaveformGraph in"=w828) -> ()  [unwired: 7 in, 1 out]
            n212 = call "drawRoi.vi"("bit depth"=w826, "ROI"=w833, "Reff image"=w821, "Whole image"=w819) -> ("size"=→"size":i32, "mean"=w825:dbl, "Image Out"=→"CCD Image":T6, "Percentile alert"=w812:bool)  [unwired: 3 in, 1 out]
            n213 = Tick Count (ms)() -> (millisecond timer value=w835:u32)
            n214 = Subtract(x=w835, y=w844) -> (x-y=w847:u32)
            n215 = Reciprocal(x=w847) -> (1/x=w846:dbl)
            n216 = call "meanAndVar.vi"("new mean value"=w825, "MEAN array in"=w816, "VAR array in"=w815) -> ("arrays stack"=→"Chart TimeSeries":dbl[][], "MEAN array out"=w814:dbl[], "VAR array out"=w813:dbl[])  [unwired: 2 in]
            n217 = Multiply(x=u32 1000 ("y"), y=w846) -> (x*y=→"Real FPS":dbl)
            n218 = property on="Reff alert" class="Bool (strict)"("Blinking"=w812) -> ()  [unwired: 2 in, 2 out]
          }
          event "take reff", "Reset reff.": Value Change {
            w851 = dbl[] [] ("RefTimeSeries")
            w850 = FALSE ("take reff")
            n219 = event-data() -> ("CtlRef"=w849:refnum<vi>)  [unwired: 1 in, 5 out]
            n220 = property class="Bool (strict)"(reference=w849) -> ("Label.Text"=w848:string)  [unwired: 1 in, 2 out]
            n221 = case shown="\"take reff\"" w848 {
              frame "Any", Default {
              }
              frame "take reff" {
                n222 = property on="CCD Image" class="ImageControl"() -> ("ROI"=→"Reff ROI":T8)  [unwired: 2 in, 2 out]
              }
            }
            n223 = local write "Reset reff."(w850) -> ()